vi "VP_RT_standard.vi"() -> ()   [LabVIEW 2015]
uses:
  State Enum.ctl
  Command Enum.ctl
  <vilib>/Platform/TimedLoop/XDataNode/timing_clust.ctl
  <vilib>/Platform/TimedLoop/XDataNode/nitl_modes.ctl
  <vilib>/Platform/TimedLoop/XDataNode/wakeup.ctl
  Data Write Control.ctl
  <vilib>/FPGAPlugInAG/cRIO-9039/niLvFpga_Open_cRIO-9039.vi
  <vilib>/rvi/interface/common/dynamic/niFpgaDynamicAddResources.vi
  <vilib>/Utility/error.llb/Error Cluster From Error Code.vi
  <vilib>/rvi/errors/niLvFpgaAdjustHostInterfaceError.vi
  <vilib>/rvi/interface/common/niFpgaWaitOnOcc.vi
  <vilib>/FPGAPlugInAG/Dynamic/niLvFpga_Reset_Dynamic.vi
  <vilib>/FPGAPlugInAG/Dynamic/niLvFpga_Abort_Dynamic.vi
  <vilib>/FPGAPlugInAG/Dynamic/niLvFpga_Close_Dynamic.vi
  <vilib>/Platform/TimedLoop/XDataNode/XDataNode.xnode
  <vilib>/rvi/interface/nirviOpenFPGA/nirviOpenFPGA.xnode
  FPGA Bitfiles/VP_NP_FPGA_Full.lvbitx
  <vilib>/rvi/interface/nirviReadWriteControl/nirviReadWriteControl.xnode
  <vilib>/rvi/interface/nirviMethod/nirviMethod.xnode
  <vilib>/rvi/interface/nirviCloseFPGA/nirviCloseFPGA.xnode
  <vilib>/Platform/TimedLoop/XDataNode/XDNodeRunTimeDep.lvlib
  <vilib>/rvi/errors/niLvFpgaMergeErrorWithErrorCode.vi
  NiFpgaLv.dll
  <vilib>/rvi/interface/Simulation/niFpgaSimulationCallBeginRW.vi
  <vilib>/rvi/Analysis/host/Public/NI_FpgaMspHost.lvlib
  <vilib>/FPGAPlugInAG/Dynamic/niLvFpga_StopFifo_Dynamic.vi
  <vilib>/FPGAPlugInAG/Dynamic/niLvFpga_ReadFifo_Dynamic.vi
  <vilib>/NI_Real-Time Target Support.lvlib
  <vilib>/FPGAPlugInAG/Dynamic/niLvFpga_ConfigureFifo_Dynamic.vi
panel:
  out "Z-Stage Input In Range?":bool=TRUE
  out "Y-Stage Input In Range?":bool=TRUE
  out "X-Stage Input In Range?":bool=TRUE
  in  "Tab Control":T1(tab)
  out "Fly Scan Complete":bool
  out "XY actual":cluster{"Array":dbl[], "Array":dbl[]}(graph)
  out "XY Ref":cluster{"Array":dbl[], "Array":dbl[]}(graph)
  out "Elements Available in FIFO":u32(graph)
  out "Elements Remaining in FIFO":u32(graph)
  out "Reference and Actual positions":cluster{"t0":dbl, dbl, dbl[][]}(graph)
  in  "Timeout FPGA FIFO1":i32=40000000
  out "FIFO Timed Out":bool
  out "stop case":bool
  in  "Datalog Cases":T2(ring)=enum."Data Log 16"
  out "FIFO Timed Out?":bool
  in  "FIFO Time Period":dbl=0.01 format="%#_13g"
  out "Number of Elements":u32=1250
  out "Datalog Rate (Hz)":dbl=25000.000000000004
  out "Elements Remaining":u32
  in  "Timeout (ms)":i32=10000
  out "Actual Depth":u32=131068416
  in  "Requested Depth":u32=131068000
  out "2iddVELO:VP:X_End_nm":dbl=2000.0
  out "2iddVELO:VP:X_Start_nm":dbl=-2000.0
  out "2iddVELO:VP:Start_Scan":bool
  out "2iddVELO:VP:Y_Start_nm":dbl=2000.0
  out "2iddVELO:VP:Y_End_nm":dbl=-2000.0
  out "2iddVELO:VP:Y_Step_Size_nm":dbl=50.0
  out "2iddVELO:VP:X_Step_Size_nm":dbl=50.0
  out "2iddVELO:VP:Trigger_Freq_Hz":dbl=1000.0
  out "2iddVELO:VP:Trig_DutyCycle_Per":dbl=99.0
  out "Iteration Duration RT Timed-Loop":i64=128
  in  "X Ramp Start (nm)":fxp<+/-,16,16>=-500.0
  in  "X Ramp End (nm)":fxp<+/-,16,16>=500.0
  in  "X Start Marker (nm)":fxp<+/-,58,25>
  in  "Y Ramp Start (nm)":fxp<+/-,16,16>=500.0
  in  "Y Ramp End (nm)":fxp<+/-,16,16>=-500.0
  in  "Y Step Size (nm)":fxp<+/-,16,16>=50.0
  in  "Y Start Marker (nm)":fxp<+/-,58,25>
  out "Fly Scan Running":bool
  out "Continue Run":bool
  out "X Ramp Period (usec)":fxp<+,24,24>=60000.0
  out "Y Ramp Period (usec)":fxp<+,24,24>=60000.0
  out "# of Hor Lines":fxp<+/-,34,18>=181.0 format="%.22g"
  in  "X Step Size (nm)":fxp<+/-,16,16>=50.0
  out "# of Points per Line":fxp<+/-,33,17>=180.0
  out "# Total Trigger Points":fxp<+/-,64,34>=32580.0
  out "sec per line":dbl=0.06
  out "line per sec (Hz)":dbl=16.666666666666668
  out "X Ramp Period DBL (usec)":dbl=60000.0 format="%#_6f"
  out "Total Scan Time (sec)":dbl=10.86
  in  "Controller Time Period (uSec)":u32=40
  in  "Controller Output Time Period (uSec)":u32=40
  in  "X Reference Time Period (uSec)":u32=40
  in  "Plant Output Time Period (uSec)":u32=40
  in  "Stop System (Careful!!)":bool
  in  "Datalog Time Period (uSec)":u32=40
  in  "Analog Input Time Period (uSec)":u32=40
  in  "Detector Trigger Time Period (uSec)":u32=40
  in  "Trigger Generation Time Period (uSec)":u32=40
  in  "Y Reference Time Period (uSec)":u32=40
  in  "Z Reference Time Period (uSec)":u32=40
  in  "Data Trigger Time Period (uSec)":u32=40
  in  "Reset All":bool
  in  "System Loop Type":enum16{"Open Loop", "Closed Loop"}(ring)
  in  "Base name":string="base_name"
  out "Trigger for Data":fxp<+/-,58,25>=1.0
  out "Data":fxp<+/-,58,25>[](array[numeric])
  out "Number of Data Strings":i32=5
  out "Mod6/DIO3":bool
  out "Mod5/DIO3":bool
  out "Mod4/DIO3":bool
  in  "Sample Z Stage Resolution (nm)":fxp<+,33,3>=0.5
  in  "Sample Y Stage Resolution (nm)":fxp<+,33,3>=0.5
  in  "Sample X Stage Resolution (nm)":fxp<+,33,3>=0.5
  in  "Optics Z Stage Resolution (nm)":fxp<+,33,3>=0.5
  in  "Optics Y Stage Resolution (nm)":fxp<+,33,3>=0.5
  in  "Optics X Stage Resolution (nm)":fxp<+,33,3>=0.5
  in  "Sample Z Reset":bool
  in  "Sample Y Reset":bool
  in  "Sample X Reset":bool
  out "Mod6/DIO2":bool
  out "Mod6/DIO1":bool
  out "Mod6/DIO0":bool=TRUE
  out "Mod5/DIO2":bool
  out "Mod5/DIO1":bool=TRUE
  out "Mod5/DIO0":bool
  out "Mod4/DIO2":bool=TRUE
  out "Mod4/DIO1":bool
  out "Mod4/DIO0":bool=TRUE
  in  "Optics Z Reset":bool
  in  "Optics Y Reset":bool
  in  "Optics X Reset":bool
  in  "Detector Trigger Lower Limit (V)":fxp<+/-,20,5>
  in  "Detector Trigger Upper Limit (V)":fxp<+/-,20,5>=5.0
  out "Detector Trigger (V)":fxp<+/-,20,5>
  out "Detector Trigger In Range?":bool=TRUE
  in  "Trigger High Period (usec)":fxp<+/-,64,45>=1250.0
  in  "Trigger Low Period (usec)":fxp<+/-,64,45>=1250.0
  in  "Trigger High Level (V)":fxp<+/-,20,5>=5.0
  in  "Trigger Low Level (V)":fxp<+/-,20,5>
  in  "Trigger Wave Generator":T3(ring)=enum."Square Wave 1"
  in  "DT Reference Amplitude (V)":fxp<+/-,40,17>=5.0
  in  "DT Reference DC Offset (V)":fxp<+/-,16,16>
  out "DT Frequency (periods/tick)":fxp<+,32,0>=7.500010542571545e-05
  out "DT Phase Offset (periods)":fxp<+,32,0>
  in  "DT Reset":bool
  out "DT Duty Cycle (periods)":fxp<+,32,0>=0.8799999998882413
  in  "DT phase offset (deg)":dbl format="%#.6g"
  in  "DT Frequency (Hz)":dbl=200.0 format="%#_6p"
  in  "DT duty cycle (%)":dbl=88.0 min=0.0 max=100.0 step=1.0
  in  "Z White Noise Seed":u32=4
  in  "Z White Noise Amplitude":u16=32767
  in  "Y White Noise Seed":u32=4
  in  "Y White Noise Amplitude":u16=32767
  in  "Z Reference Reset":bool
  in  "Y Reference Reset":bool
  in  "X Reference Reset":bool
  in  "Z Reference Wave Selection":T4(ring)=enum."Sine Wave"
  in  "X Reference Wave Selection":T5(ring)=enum."Custom Up Down Ramp"
  in  "Y Reference Wave Selection":T6(ring)=enum."Custom Ramp Wave"
  out "Z phase offset (periods)":fxp<+,32,0>
  out "Z frequency (periods/tick)":fxp<+,32,0>=1.25030055642128e-07 format="%.32g"
  in  "Z phase offset (deg)":dbl format="%#.6g"
  in  "Z frequency (Hz)":dbl=5.0 format="%#_6p"
  out "Y phase offset (periods)":fxp<+,32,0>
  out "Y frequency (periods/tick)":fxp<+,32,0>=5.005858838558197e-08 format="%.32g"
  in  "Y phase offset (deg)":dbl format="%#.6g"
  in  "Y frequency (Hz)":dbl=2.0 format="%#_6p"
  out "Z Stage Reference (nm)":fxp<+/-,58,25>
  out "Y Stage Reference (nm)":fxp<+/-,58,25>
  out "X Stage Reference (nm)":fxp<+/-,58,25>
  in  "X White Noise Seed":u32=4
  in  "X White Noise Amplitude":u16=32767
  in  "Z Reference DC Offset (nm)":fxp<+/-,15,15>
  in  "Y Reference DC Offset (nm)":fxp<+/-,16,16>
  in  "X Reference DC Offset (nm)":fxp<+/-,16,16>
  in  "Z Reference Amplitude (nm)":fxp<+/-,40,17>
  in  "Y Reference Amplitude (nm)":fxp<+/-,40,17>=100.0
  in  "X Reference Amplitude (nm)":fxp<+/-,40,17>=100.0
  out "X phase offset (periods)":fxp<+,32,0>
  out "X frequency (periods/tick)":fxp<+,32,0>=1.25030055642128e-07 format="%.32g"
  in  "X phase offset (deg)":dbl format="%#.6g"
  in  "X frequency (Hz)":dbl=5.0 format="%#_6p"
  in  "Scaling mV to V":fxp<+,33,10>=0.001000046730041504
  out "Heartbeat":bool=TRUE
  in  "System command":T7
  in  "Execute":bool
  out "Last Command Executed":T7
  in  "Optics and or Sample Stage":T8(ring)
  out "2iddVELO:VP:Fly_Scan":bool
  out "Remote Mode":bool
  in  "Fly Scan":bool
  in  "Local_Lock":bool
  out "Snake Scan Reference FPGA or EPICS":enum16{"FPGA Snake Scan", "EPICS Snake Scan"}(ring)
  out "Output filename":string
  out "Output path":path
  out "FPGA state":T9(ring)
  in  "cRIO data dir":string="/home/lvuser/natinst/data"
  out "RT Main Loop State":T10
  out "cRIO path":path
  out "Trigger Frequency (Hz)":dbl
  out "Trigger Duty Cycle (%)":dbl
  in  "Z-Stage Scaling Direction":fxp<+/-,3,3>=-1.0
  in  "Y-Stage Scaling Direction":fxp<+/-,3,3>=-1.0
  in  "Mod 3 AI2 V to nm Scaling":fxp<+,47,18>=1000.0
  in  "Mod 3 AI1 V to nm Scaling":fxp<+,47,18>=1000.0
  in  "Mod 3 AI0 V to nm Scaling":fxp<+,47,18>=1000.0
  out "PI Z-Stage Input (V)":fxp<+/-,20,5>=-0.000732421875
  out "PI Y-Stage Input (V)":fxp<+/-,20,5>=0.005584716796875
  out "PI X-Stage Input (V)":fxp<+/-,20,5>=-0.00311279296875
  in  "Z-Stage nm to V Scaling":fxp<+/-,32,12>=0.0005397796630859375
  in  "Y-Stage nm to V Scaling":fxp<+/-,32,12>=0.0014200210571289062
  in  "X-Stage Scaling Direction":fxp<+/-,3,3>=-1.0
  in  "X-Stage nm to V Scaling":fxp<+/-,32,12>=0.0005359649658203125
  in  "Controller Output Lower Limit":fxp<+/-,20,5>=-5.0
  in  "Controller Output Upper Limit":fxp<+/-,20,5>=5.0
  in  "FPGA Wait Timer (ms)":u16=50
  in  "Pre-Scan pause (ms)":u32=250
  in  "Readback Loop time between iterations (ms)":u32=10
  out "Measured Datalog Time Period (Ticks)":u32=1600
  out "Measured Datalog Loop Rate (secs)":dbl=3.9999999999999996e-05
  out "Measured Datalog Loop Rate (kHz)":dbl=25.000000000000004
  out "Measured Counter Loop Rate (secs)":dbl
  out "Measured Counter Loop Rate (MHz)":dbl=inf
  out "Measured X Reference Loop Rate (secs)":dbl=3.9999999999999996e-05
  out "Measured X Reference Loop Rate (kHz)":dbl=25.000000000000004
  out "Measured X Reference Time Period (Ticks)":u32=1600
  out "Measured Controller Loop Rate (kHz)":dbl=25.000000000000004
  out "Measured Controller Output Loop Rate (secs)":dbl=3.9999999999999996e-05
  out "Measured Controller Output Loop Rate (kHz)":dbl=25.000000000000004
  out "Measured Plant Output Loop Rate (secs)":dbl=3.9999999999999996e-05
  out "Measured Plant Output Loop Rate (kHz)":dbl=25.000000000000004
  out "Measured Controller Loop Rate (secs)":dbl=3.9999999999999996e-05
  out "Measured Controller Time Period (Ticks)":u32=1600
  out "Datalog Time Period (sec)":dbl=3.9999999999999996e-05
  out "Measured Controller Output Time Period (Ticks)":u32=1600
  out "Measured Plant Output Time Period (Ticks)":u32=1600
  out "Measured Counter Time Period (Ticks)":u32
  out "32 bit Count Optics X":i32
  out "32 bit Count Optics  Y":i32
  out "32 bit Count Optics  Z":i32
  out "32 bit Count Sample X":i32
  out "32 bit Count Sample  Y":i32=2
  out "32 bit Count Sample  Z":i32=-4
  out "Optics X Stage Displacement (nm)":fxp<+/-,58,25>=-1.0
  out "Optics Y Stage Displacement (nm)":fxp<+/-,58,25>
  out "Optics Z Stage Displacement (nm)":fxp<+/-,58,25>
  out "Sample X Stage Displacement (nm)":fxp<+/-,58,25>=-0.5
  out "Sample Y Stage Displacement (nm)":fxp<+/-,58,25>=1.5
  out "Sample Z Stage Displacement (nm)":fxp<+/-,58,25>=-1.0
  out "Measured Analog Input Time Period (Ticks)":u32=1600
  out "Measured Analog Input Loop Rate (secs)":dbl=3.9999999999999996e-05
  out "Measured Analog Input Loop Rate (kHz)":dbl=25.000000000000004
  out "Measured Detector Trigger Time Period (Ticks)":u32=1600
  out "Measured Trigger Gen Time Period (Ticks)":u32=1600
  out "Measured Y Reference Time Period (Ticks)":u32=1600
  out "Measured Z Reference Time Period (Ticks)":u32=1600
  out "Measured Y Reference Loop Rate (secs)":dbl=3.9999999999999996e-05
  out "Measured Y Reference Loop Rate (kHz)":dbl=25.000000000000004
  out "Measured Z Reference Loop Rate (secs)":dbl=3.9999999999999996e-05
  out "Measured Z Reference Loop Rate (kHz)":dbl=25.000000000000004
  out "Measured Data Trigger Time Period (Ticks)":u32=1600
  in  "file path soscoeff_xx1":path=path "C:/ni-rt/startup/2 ID D/Kxx/Kxx_1_Gxx_md_40us/Kxx_1_Gxx_matched_dow_16ord_mVpnm_cd8a3_AvTio9_X5nm_500pm_all_40us_soscof_xx1.mat"
  in  "file path sos gain SF Controller_xx1":path=path "C:/ni-rt/startup/2 ID D/Kxx/Kxx_1_Gxx_md_40us/Kxx_1_Gxx_matched_dow_16ord_mVpnm_cd8a3_AvTio9_X5nm_500pm_all_40us_soscof_xx2.mat"
  in  "file path soscoeff_yy1":path=path "C:/ni-rt/startup/2 ID D/Kyy/Kyy_trial_1_Gyy_md_40us/Kyy_trial_1_Gyy_matched_dow_8ord_mVpnm_cd8a3_AvTio9_Y5nm_500pm_all_40us_soscof_yy1.mat"
  in  "file path sos gain SF Controller_yy1":path=path "C:/ni-rt/startup/2 ID D/Kyy/Kyy_trial_1_Gyy_md_40us/Kyy_trial_1_Gyy_matched_dow_8ord_mVpnm_cd8a3_AvTio9_Y5nm_500pm_all_40us_soscof_yy2.mat"
  in  "file path soscoeff_zz1":path=path "C:/ni-rt/startup/2 ID D/Kzz/Kzz_1_Gzz_md_40us/Kzz_1_Gzz_matched_dow_29ord_mVpnm_cd8a3_AvTio9_Z5nm_500pm_all_40us_soscof_zz1.mat"
  in  "file path sos gain SF Controller_zz1":path=path "C:/ni-rt/startup/2 ID D/Kzz/Kzz_1_Gzz_md_40us/Kzz_1_Gzz_matched_dow_29ord_mVpnm_cd8a3_AvTio9_Z5nm_500pm_all_40us_soscof_zz2.mat"
  in  "file path soscoeff_yx1":path=path "C:/ni-rt/startup/2 ID D/Kxx/Kxx_1_Gxx_md_40us/allzero_mVpnm_XX_XY_XZ_YX_YY_YZ_ZX_ZY_ZZ_woffst_soscoeff1.mat"
  in  "file path sos gain SF Controller_yx1":path=path "C:/ni-rt/startup/2 ID D/Kxx/Kxx_1_Gxx_md_40us/allzero_mVpnm_XX_XY_XZ_YX_YY_YZ_ZX_ZY_ZZ_woffst_soscoeff2.mat"
  in  "file path soscoeff_zx1":path=path "C:/ni-rt/startup/2 ID D/Kxx/Kxx_1_Gxx_md_40us/allzero_mVpnm_XX_XY_XZ_YX_YY_YZ_ZX_ZY_ZZ_woffst_soscoeff1.mat"
  in  "file path sos gain SF Controller_zx1":path=path "C:/ni-rt/startup/2 ID D/Kxx/Kxx_1_Gxx_md_40us/allzero_mVpnm_XX_XY_XZ_YX_YY_YZ_ZX_ZY_ZZ_woffst_soscoeff2.mat"
  in  "file path soscoeff_xy1":path=path "C:/ni-rt/startup/2 ID D/Kxx/Kxx_1_Gxx_md_40us/allzero_mVpnm_XX_XY_XZ_YX_YY_YZ_ZX_ZY_ZZ_woffst_soscoeff1.mat"
  in  "file path sos gain SF Controller_xy1":path=path "C:/ni-rt/startup/2 ID D/Kxx/Kxx_1_Gxx_md_40us/allzero_mVpnm_XX_XY_XZ_YX_YY_YZ_ZX_ZY_ZZ_woffst_soscoeff2.mat"
  in  "file path soscoeff_zy1":path=path "C:/ni-rt/startup/2 ID D/Kxx/Kxx_1_Gxx_md_40us/allzero_mVpnm_XX_XY_XZ_YX_YY_YZ_ZX_ZY_ZZ_woffst_soscoeff1.mat"
  in  "file path sos gain SF Controller_zy1":path=path "C:/ni-rt/startup/2 ID D/Kxx/Kxx_1_Gxx_md_40us/allzero_mVpnm_XX_XY_XZ_YX_YY_YZ_ZX_ZY_ZZ_woffst_soscoeff2.mat"
  in  "file path soscoeff_xz1":path=path "C:/ni-rt/startup/2 ID D/Kxx/Kxx_1_Gxx_md_40us/allzero_mVpnm_XX_XY_XZ_YX_YY_YZ_ZX_ZY_ZZ_woffst_soscoeff1.mat"
  in  "file path sos gain SF Controller_xz1":path=path "C:/ni-rt/startup/2 ID D/Kxx/Kxx_1_Gxx_md_40us/allzero_mVpnm_XX_XY_XZ_YX_YY_YZ_ZX_ZY_ZZ_woffst_soscoeff2.mat"
  in  "file path soscoeff_yz1":path=path "C:/ni-rt/startup/2 ID D/Kxx/Kxx_1_Gxx_md_40us/allzero_mVpnm_XX_XY_XZ_YX_YY_YZ_ZX_ZY_ZZ_woffst_soscoeff1.mat"
  in  "file path sos gain SF Controller_yz1":path=path "C:/ni-rt/startup/2 ID D/Kxx/Kxx_1_Gxx_md_40us/allzero_mVpnm_XX_XY_XZ_YX_YY_YZ_ZX_ZY_ZZ_woffst_soscoeff2.mat"
  out "-a01(2) xx1c":fxp<+/-,64,9>[](array[numeric])=[0.637785025840232, 0.9924182654286198, 1.8461027816316544, 0.8635404845716299, 1.0670555456779864, 1.6350703383821101, 1.6323955588345012, 1.1102241390539636, 0.0, 0.0, 0.0, 0.0, 0.0, 0.0, 0.0, 0.0, 0.0, 0.0, 0.0, 0.0]
  out "-a02(2) xx1c":fxp<+/-,64,9>[](array[numeric])=[-0.999855815746439, -0.9676991072632725, -0.9642268720534838, -0.9446498323360957, -0.9442808087139987, -0.7547983908829242, -0.6690016013017409, -0.11027986125857198, 0.0, 0.0, 0.0, 0.0, 0.0, 0.0, 0.0, 0.0, 0.0, 0.0, 0.0, 0.0]
  out "b01(2) xx1c":fxp<+/-,64,9>[](array[numeric])=[-0.6378105164532328, -1.0062332697665268, -1.8762916543815855, -0.8616288879491845, -1.0856571140792324, -1.6862585929720944, -1.743591709663851, -0.6129835805090948, 0.0, 0.0, 0.0, 0.0, 0.0, 0.0, 0.0, 0.0, 0.0, 0.0, 0.0, 0.0]
  out "b02(2) xx1c":fxp<+/-,64,9>[](array[numeric])=[0.9999102047610771, 0.9971375605901365, 0.9926840301018772, 0.9509648854364836, 0.9563369558920378, 0.7818900462139817, 0.7642575436257291, 3.0531133177191805e-16, 0.0, 0.0, 0.0, 0.0, 0.0, 0.0, 0.0, 0.0, 0.0, 0.0, 0.0, 0.0]
  out "sos gain SF Controller xx1c":fxp<+/-,42,9>=-0.1625035791657865
  out "-a01(2) yy1c":fxp<+/-,64,9>[](array[numeric])=[1.8740229377643998, 1.3096977339382483, 1.7453886241944765, 0.2668895009727739, 0.0, 0.0, 0.0, 0.0, 0.0, 0.0, 0.0, 0.0, 0.0, 0.0, 0.0, 0.0, 0.0, 0.0, 0.0, 0.0]
  out "-a02(2) yy1c":fxp<+/-,64,9>[](array[numeric])=[-0.9732703278433918, -0.5194903821190732, -0.7453924481836136, -2.7755575615628914e-17, 0.0, 0.0, 0.0, 0.0, 0.0, 0.0, 0.0, 0.0, 0.0, 0.0, 0.0, 0.0, 0.0, 0.0, 0.0, 0.0]
  out "b01(2) yy1c":fxp<+/-,64,9>[](array[numeric])=[-1.8979173162254057, -1.8463149313261074, -1.7151162246453355, -0.006444279582847878, 0.0, 0.0, 0.0, 0.0, 0.0, 0.0, 0.0, 0.0, 0.0, 0.0, 0.0, 0.0, 0.0, 0.0, 0.0, 0.0]
  out "b02(2) yy1c":fxp<+/-,64,9>[](array[numeric])=[0.9969084979865663, 0.9421233904433339, 0.7362048104846675, 0.0, 0.0, 0.0, 0.0, 0.0, 0.0, 0.0, 0.0, 0.0, 0.0, 0.0, 0.0, 0.0, 0.0, 0.0, 0.0, 0.0]
  out "sos gain SF Controller yy1c":fxp<+/-,42,9>=-1.480983349494636
  out "-a01(2) zz1c":fxp<+/-,64,9>[](array[numeric])=[0.6242394224317618, 1.8967038692417004, 0.6659160318030806, 1.7792660019034106, 1.6870099721477447, 0.6417945190222861, 1.4838029149808185, 1.8456549628851837, 1.2189509782386598, 0.9933314517253298, 1.0158915520299678, 0.8863484387433826, 0.026837806879254994, 1.8269783715122585, 0.22448441435364225, 0.0, 0.0, 0.0, 0.0, 0.0]
  out "-a02(2) zz1c":fxp<+/-,64,9>[](array[numeric])=[-0.9983298461163967, -0.9972287452752734, -0.995744457243837, -0.9947210838396919, -0.9925914602095722, -0.9920974045271405, -0.9881915357970101, -0.9800069383591395, -0.9760641145386646, -0.9508624135515895, -0.9242774595356998, -0.655945641403593, -0.008661844724279444, -0.8269827070369743, 0.0, 0.0, 0.0, 0.0, 0.0, 0.0]
  out "b01(2) zz1c":fxp<+/-,64,9>[](array[numeric])=[-0.6245671059510156, -1.897930093390194, -0.6670970070931089, -1.7670265604573054, -1.6833314913922348, -0.6327437892303018, -1.5025901530730128, -1.8636454269915796, -1.1210694827766767, -0.9982206064398196, -1.0326369335418408, -1.1342635673267367, -1.6852506306166828, -0.9843740162364313, -1.7208456881689926e-15, 0.0, 0.0, 0.0, 0.0, 0.0]
  out "b02(2) zz1c":fxp<+/-,64,9>[](array[numeric])=[0.9973135069419645, 0.9951302056171929, 0.9993435624612031, 0.9919371251860779, 0.994931751453586, 0.9881092761723503, 0.9884874399279107, 0.9977145546300196, 0.9725302934743221, 0.9855561672767964, 0.9893454712398023, 0.846212786518208, 0.7855598927779743, 0.0978075435519738, 0.0, 0.0, 0.0, 0.0, 0.0, 0.0]
  out "sos gain SF Controller zz1c":fxp<+/-,42,9>=-0.1988595259608701
  out "-a01(2) yx1c":fxp<+/-,64,9>[](array[numeric])
  out "-a02(2) yx1c":fxp<+/-,64,9>[](array[numeric])
  out "b01(2) yx1c":fxp<+/-,64,9>[](array[numeric])
  out "b02(2) yx1c":fxp<+/-,64,9>[](array[numeric])
  out "sos gain SF Controller yx1c":fxp<+/-,42,9>
  out "-a01(2) zx1c":fxp<+/-,64,9>[](array[numeric])
  out "-a02(2) zx1c":fxp<+/-,64,9>[](array[numeric])
  out "b01(2) zx1c":fxp<+/-,64,9>[](array[numeric])
  out "b02(2) zx1c":fxp<+/-,64,9>[](array[numeric])
  out "sos gain SF Controller zx1c":fxp<+/-,42,9>
  out "-a01(2) xy1c":fxp<+/-,64,9>[](array[numeric])
  out "-a02(2) xy1c":fxp<+/-,64,9>[](array[numeric])
  out "b01(2) xy1c":fxp<+/-,64,9>[](array[numeric])
  out "b02(2) xy1c":fxp<+/-,64,9>[](array[numeric])
  out "sos gain SF Controller xy1c":fxp<+/-,42,9>
  out "-a01(2) zy1c":fxp<+/-,64,9>[](array[numeric])
  out "-a02(2) zy1c":fxp<+/-,64,9>[](array[numeric])
  out "b01(2) zy1c":fxp<+/-,64,9>[](array[numeric])
  out "b02(2) zy1c":fxp<+/-,64,9>[](array[numeric])
  out "sos gain SF Controller zy1c":fxp<+/-,42,9>
  out "-a01(2) xz1c":fxp<+/-,64,9>[](array[numeric])
  out "-a02(2) xz1c":fxp<+/-,64,9>[](array[numeric])
  out "b01(2) xz1c":fxp<+/-,64,9>[](array[numeric])
  out "b02(2) xz1c":fxp<+/-,64,9>[](array[numeric])
  out "sos gain SF Controller xz1c":fxp<+/-,42,9>
  out "-a01(2) yz1c":fxp<+/-,64,9>[](array[numeric])
  out "-a02(2) yz1c":fxp<+/-,64,9>[](array[numeric])
  out "b01(2) yz1c":fxp<+/-,64,9>[](array[numeric])
  out "b02(2) yz1c":fxp<+/-,64,9>[](array[numeric])
  out "sos gain SF Controller yz1c":fxp<+/-,42,9>
  out "error out (Sig Gen)":errorcluster
  out "FPGA error monitor":errorcluster
  out "FPGA end run error":errorcluster
  out "Timed Loop (end error)":errorcluster
  out "error out (Sig Gen) 2":errorcluster
  out "error out (Sig Gen) 3":errorcluster
  out "error out (Sig Gen) 4":errorcluster
  out "Main Loop error":errorcluster
  out "Main Loop Iterations":i32
  out "RT error":errorcluster
  out "EPICS comms error":errorcluster
  out "Readback error":errorcluster
  out "FPGA wait error":errorcluster
  out "Coeff file import error":errorcluster
  out "Readback loop Iterations":i32
  out "Command Loop Iterations":i32
  out "Heartbeat Loop Iterations":i32
  out "Reduced Array of States":T10[](array[typedef])
  out "XY Graph 3":cluster{"Array":dbl[], "Array":dbl[]}(graph)
  out "XY Graph 4":cluster{"Array":dbl[], "Array":dbl[]}(graph)
  out "2iddVELO:VP:cRIO_Command":string
  out "2iddVELO:VP:Controller_Type":string
  out "2iddVELO:VP:Scan_Type":string
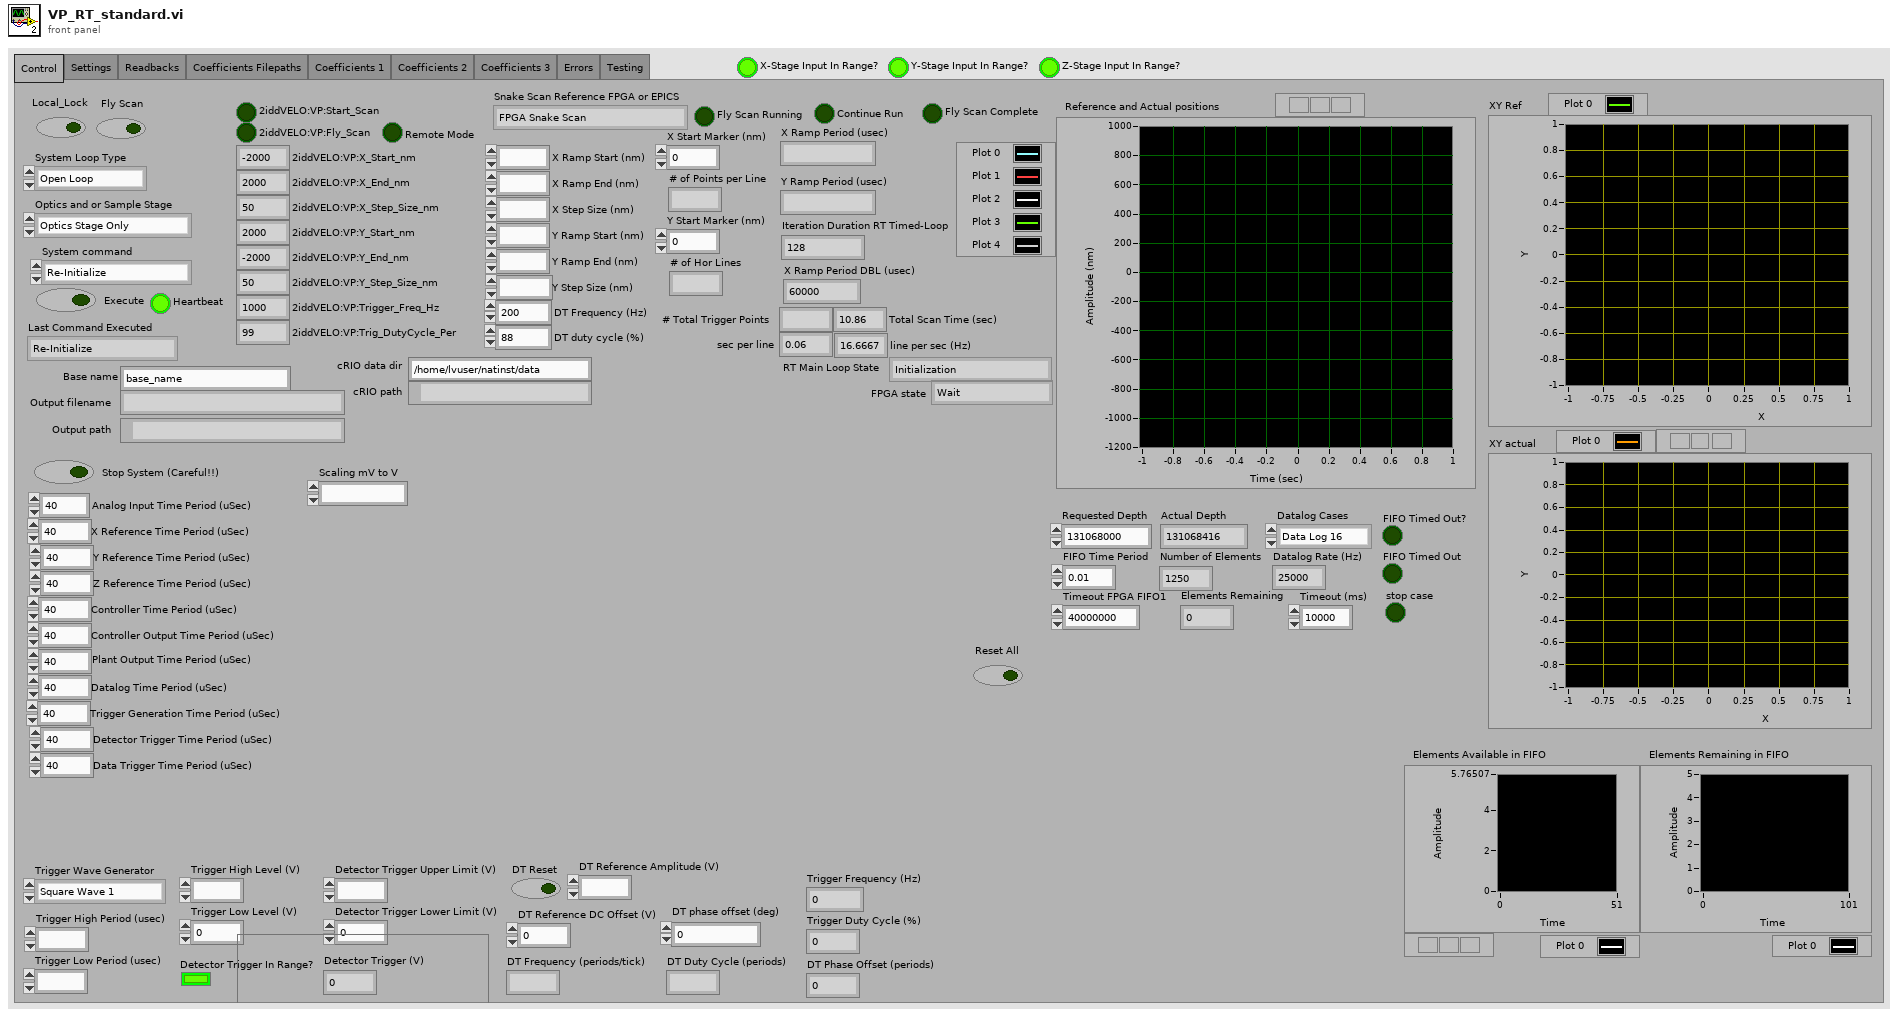
[diagram p1: front panel]
types:
  T1 = enum32{"Control", "Settings", "Readbacks", "Coefficients Filepaths", "Coefficients 1", "Coefficients 2", "Coefficients 3", "Errors", "Testing"}
  T2 = enum16{"Data Log 1", "Data Log 2", "Data Log 3", "Data Log 4", "Data Log 5", "Data Log 6", "Data Log 7", "Data Log 8", "Data Log 9", "Data Log 10", "Data Log 11", "Data Log 12", "Data Log 13", "Data Log 14", "Data Log 15", "Data Log 16"}
  T3 = enum16{"Custom Square Wave ", "Square Wave 1", "Square Wave 2"}
  T4 = enum16{"Constant", "Sine Wave", "Sawtooth Wave", "Square Wave", "Filtered White Noise"}
  T5 = enum16{"Constant", "Sine Wave", "Custom Up Down Ramp", "Filtered White Noise"}
  T6 = enum16{"Constant", "Sine Wave", "Custom Ramp Wave", "Filtered White Noise"}
  T7 = typedef "Command Enum.ctl" = enum16{"Re-Initialize ", "Update Scan Settings", "Scan", "Stop Scan", "Restart FPGA", "Stop System"}
  T8 = enum16{"Optics Stage Only", "Optics and Sample Stage"}
  T9 = enum16{"Wait", "Start Run", "Run", "End Run", "Shutdown"}
  T10 = typedef "State Enum.ctl" = enum16{"Initialization", "Import Controller coeffs", "Update Controller Info", "Wait", "Update Reference Info", "Update Detector Trigger Info", "Update Datalog Info", "Check FPGA Status", "Pre-Scan", "Start Scan", "Scanning", "End Scan", "Restart FPGA", "Stop FPGA"}
  T11 = typedef "XDNodeRunTimeDep.lvlib/timing_clust.ctl" = cluster{"Expected End [f-1]":u64, "Actual End [f-1]":u64, "Finished Late? [f-1]":bool, "Expected End [i-1]":u64, "Actual End [i-1]":u64, "Finished Late? [i-1]":bool, "Expected Start [i]":u64, "Actual Start [i]":u64, "Expected Start [f]":u64, "Actual Start [f]":u64, "Source Name":string, "Structure Name":string, "Period":i64, "Deadline":i64, "Offset":i64, "Start":i64, "Priority":i32, "Timeout":i32, "Mode":T12, "Wakeup Reason":T13, "Error":errorcluster, "Source Type":string, "Secondary Source Type":string, "Global End Time":u64, "Global Start Time":u64, "Frame Duration":u64, "Iteration Duration":u64, "Assigned CPU":i32, "I/O Scan Engine Mode":u32}
  T12 = typedef "XDNodeRunTimeDep.lvlib/nitl_modes.ctl" = enum32{"No Change", "Process missed periods, maintain original phase", "Discard missed periods, maintain original phase", "Process missed periods, ignore original phase", "Discard missed periods, ignore original phase"}
  T13 = typedef "XDNodeRunTimeDep.lvlib/wakeup.ctl" = enum32{"Normal", "Aborted", "Asynchronous wakeup", "Timing source error", "Timed loop error", "Timeout"}
  T14 = typedef "Data Write Control.ctl" = enum16{"Initialize", "Read", "Write", "Close"}
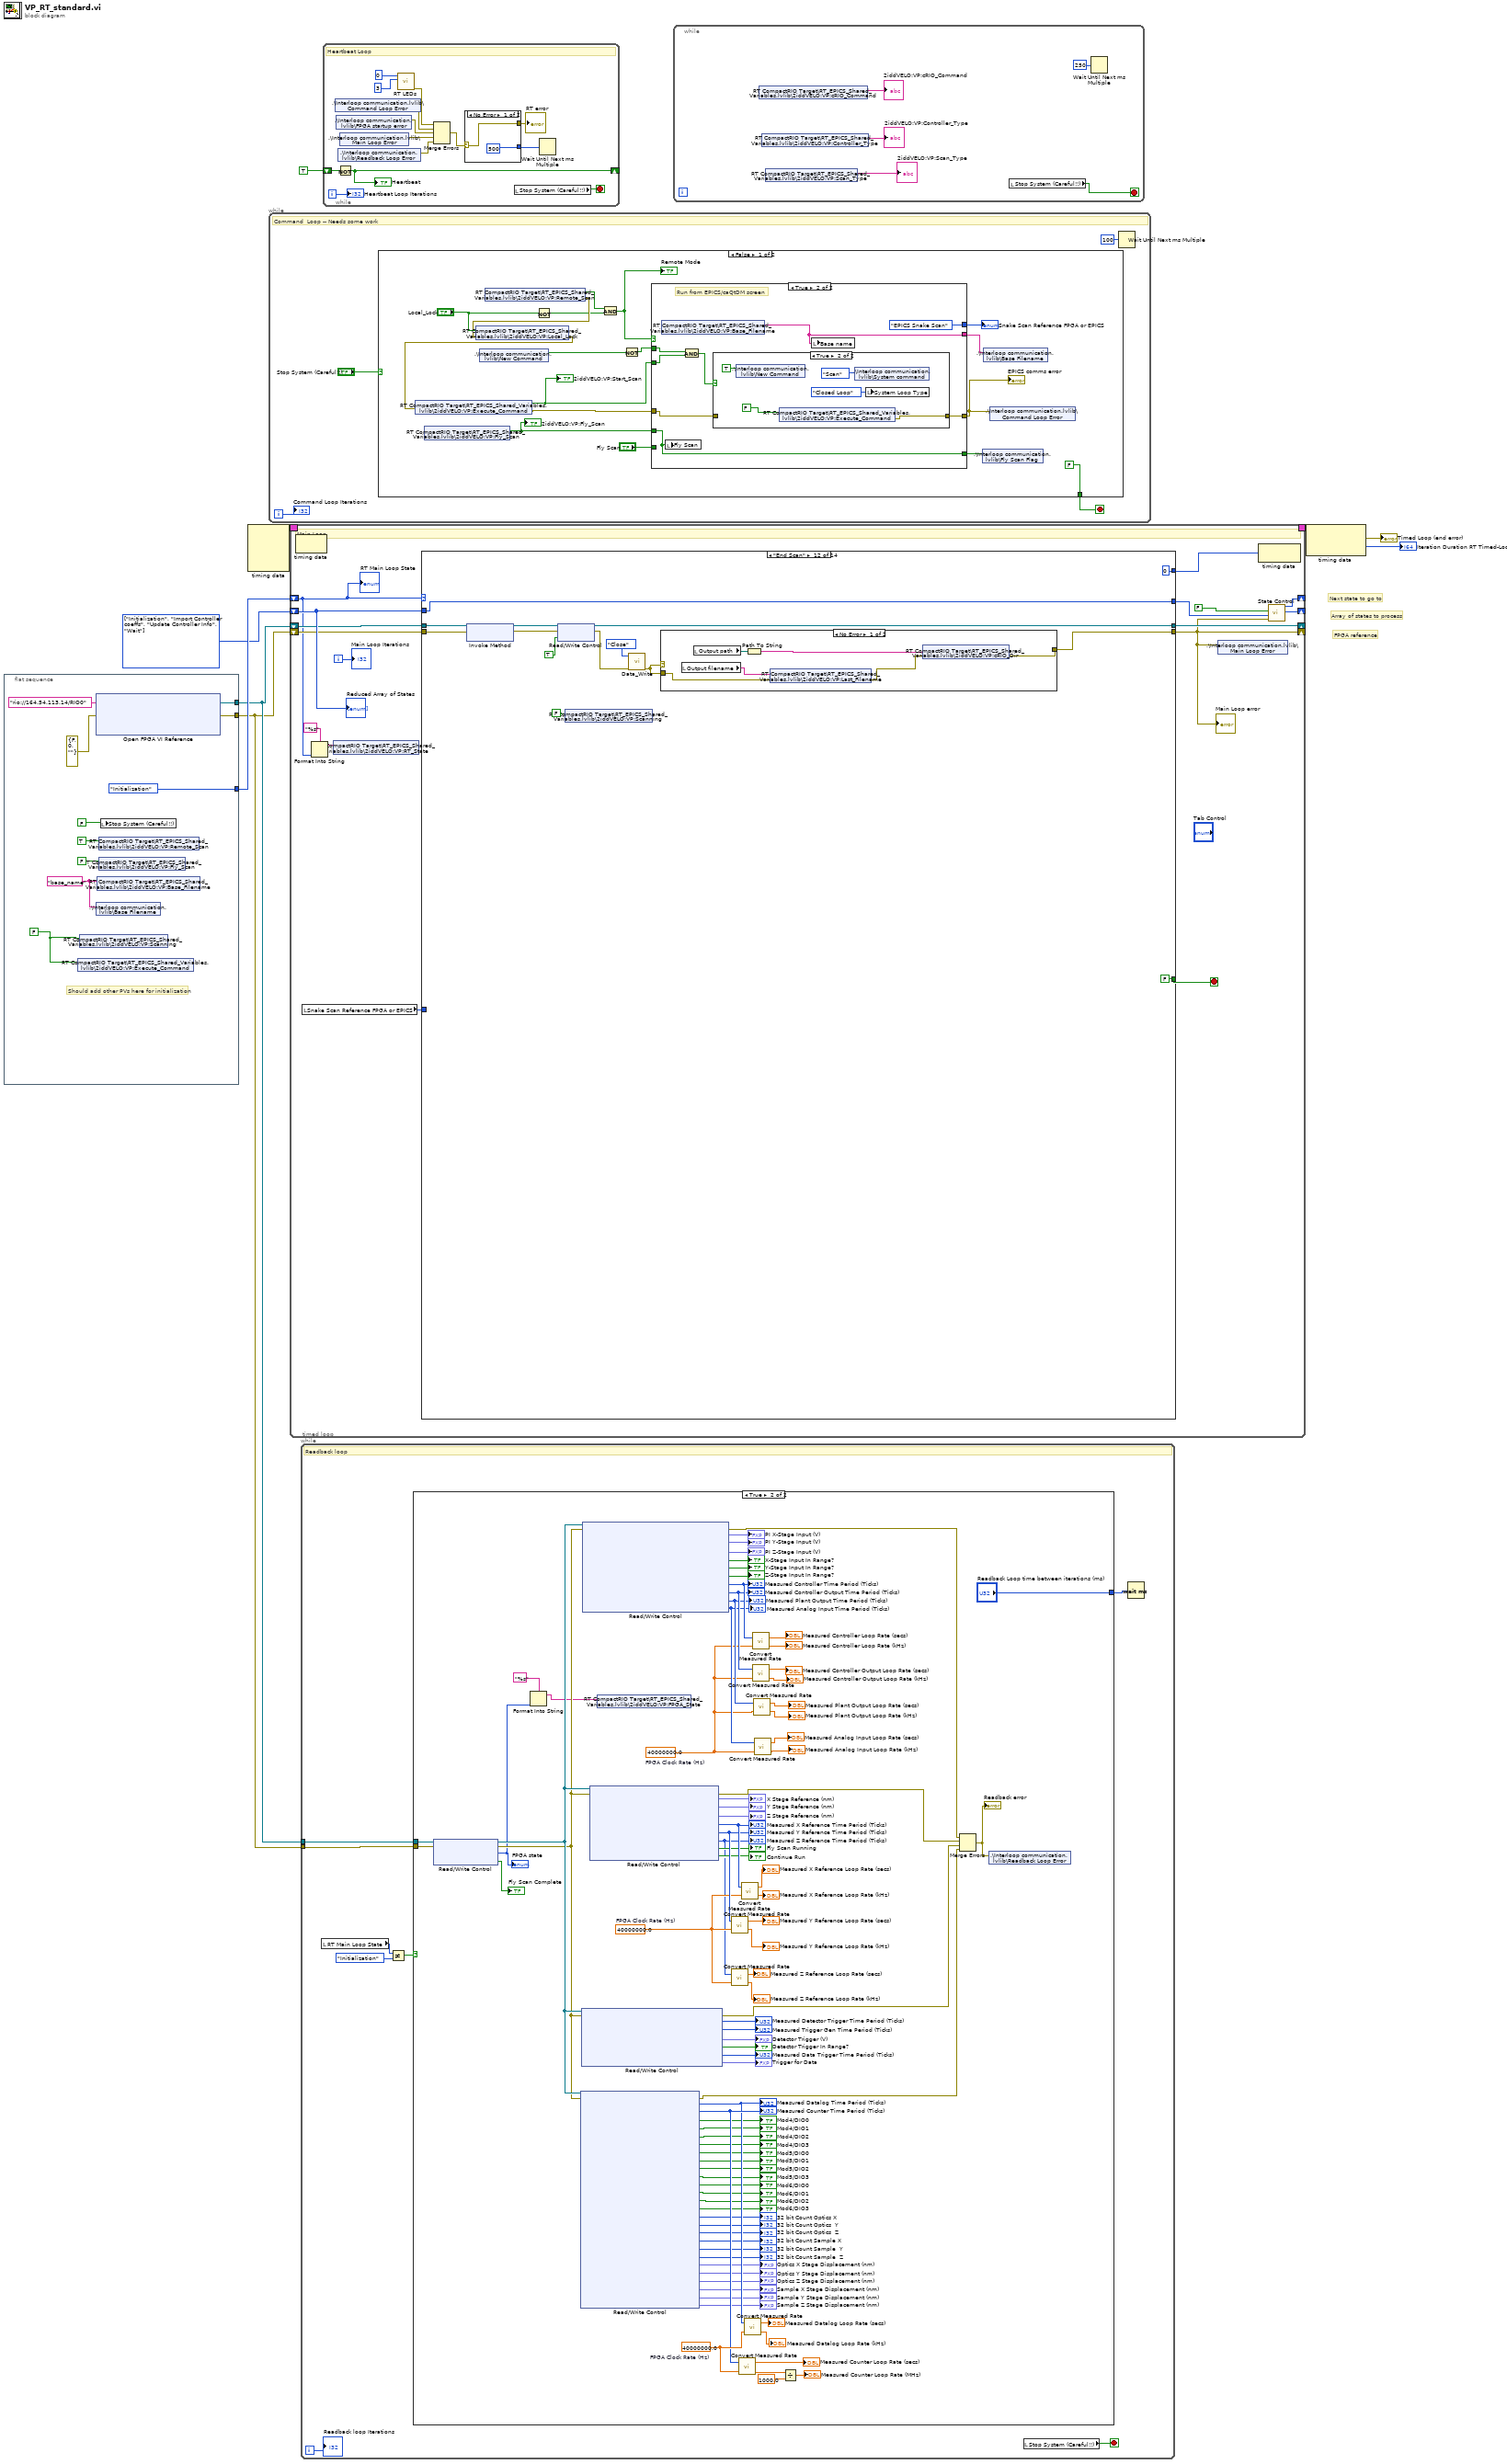
[diagram p0: block diagram]
diagram:
  w3 = T10[] [enum."Initialization", enum."Import Controller coeffs", enum."Update Controller Info", enum."Wait"] items=["Initialization", "Import Controller coeffs", "Update Controller Info", "Wait", "Update Reference Info", "Update Detector Trigger Info", "Update Datalog Info", "Check FPGA Status", "Pre-Scan", "Start Scan", "Scanning", "End Scan", "Restart FPGA", "Stop FPGA"] ("Reduced Array of States")
  # "FPGA reference"
  # "Array of states to process"
  # "Next state to go to"
  n1 = flat-sequence {
    tunnel: [State_Enum."Initialization" ("States")] -> w4
    tunnel: [w16] -> w1
    tunnel: [w15] -> w2
    frame #0 {
      w10 = FALSE ("Start_Scan")
      w13 = "base_name" ("Base_Filename")
      # "Should add other PVs here for initialization"
      n2 = shared-variable "RT CompactRIO Target\\RT_EPICS_Shared_Variables.lvlib\\2iddVELO:VP:Execute_Command"(w10) -> ()  [unwired: 1 in, 1 out]
      n3 = shared-variable "RT CompactRIO Target\\RT_EPICS_Shared_Variables.lvlib\\2iddVELO:VP:Scanning"(w10) -> ()  [unwired: 1 in, 1 out]
      n4 = xnode ("Open FPGA VI Reference")("error in"=errorcluster {"status"=FALSE, "code"=0, "source"=""} ("error constant"), "resource name"=tag "rio://164.54.113.14/RIO0") -> ("FPGA VI Reference Out"=w15:refnum<k20>, "error out"=w16:errorcluster)
      n5 = shared-variable ".\\Interloop communication.lvlib\\Base Filename"(w13) -> ()  [unwired: 1 in, 1 out]
      n6 = shared-variable "RT CompactRIO Target\\RT_EPICS_Shared_Variables.lvlib\\2iddVELO:VP:Base_Filename"(w13) -> ()  [unwired: 1 in, 1 out]
      n7 = shared-variable "RT CompactRIO Target\\RT_EPICS_Shared_Variables.lvlib\\2iddVELO:VP:Remote_Scan"(TRUE ("Remote_Scan")) -> ()  [unwired: 1 in, 1 out]
      n8 = shared-variable "RT CompactRIO Target\\RT_EPICS_Shared_Variables.lvlib\\2iddVELO:VP:Fly_Scan"(FALSE ("Fly_Scan")) -> ()  [unwired: 1 in, 1 out]
      n9 = local write "Stop System (Careful!!)"(FALSE ("Stop")) -> ()
    }
  }
  n10 = node-c288() -> (w9:T11)  [unwired: 4 in]
  n11 = while {
    i -> [w20]
    stop <- w21 stop-if-true
    # "Command  Loop -- Needs some work"
    n12 = case shown="False" "Stop System (Careful!!)" {
      tunnel: [FALSE TRUE] -> w21
      frame False {
        n13 = shared-variable "RT CompactRIO Target\\RT_EPICS_Shared_Variables.lvlib\\2iddVELO:VP:Fly_Scan"() -> (w29:bool)  [unwired: 1 in, 1 out]
        "2iddVELO:VP:Fly_Scan" <- w29
        n14 = shared-variable ".\\Interloop communication.lvlib\\New Command"() -> (w40:bool)  [unwired: 1 in, 1 out]
        n15 = shared-variable "RT CompactRIO Target\\RT_EPICS_Shared_Variables.lvlib\\2iddVELO:VP:Remote_Scan"() -> (w36:bool, error out=w34:errorcluster)  [unwired: 1 in]
        n16 = shared-variable "RT CompactRIO Target\\RT_EPICS_Shared_Variables.lvlib\\2iddVELO:VP:Local_Lock"("Local_Lock", error in=w34) -> (error out=w26:errorcluster)
        n17 = shared-variable "RT CompactRIO Target\\RT_EPICS_Shared_Variables.lvlib\\2iddVELO:VP:Execute_Command"(error in=w26) -> (w25:bool, error out=w24:errorcluster)
        "2iddVELO:VP:Start_Scan" <- w25
        n18 = Not(x="Local_Lock") -> (.not. x?=w31:bool)
        n19 = And(x=w36, y=w31) -> (x .and. y?=w37:bool)
        "Remote Mode" <- w37
        n20 = Not(x=w40) -> (.not. x?=w39:bool)
        n21 = case shown="True" w37 {
          tunnel: w25 -> [_ w57]
          tunnel: w39 -> [w48 w58]
          tunnel: [enum16{"FPGA Snake Scan", "EPICS Snake Scan"}."FPGA Snake Scan" ("Snake Scan Reference FPGA or EPICS") enum16{"FPGA Snake Scan", "EPICS Snake Scan"}."EPICS Snake Scan" ("Snake Scan Reference FPGA or EPICS")] -> w38
          tunnel: w24 -> [w42 w53]
          tunnel: [w41 w55] -> w33
          tunnel: ["Base name" w54] -> w30
          tunnel: w29 -> [_ w52]
          tunnel: [w43 w52] -> w28
          tunnel: "Fly Scan" -> [w43 _]
          frame False {
            # "Run in local mode"
            n22 = And(x="Execute", y=w48) -> (x .and. y?=w45:bool)
            n23 = shared-variable "RT CompactRIO Target\\RT_EPICS_Shared_Variables.lvlib\\2iddVELO:VP:Fly_Scan"(w43, error in=w42) -> (error out=w41:errorcluster)
            n24 = case shown="True" w45 {
              frame False {
              }
              frame True {
                n25 = shared-variable ".\\Interloop communication.lvlib\\New Command"(TRUE ("New Command")) -> ()  [unwired: 1 in, 1 out]
                n26 = shared-variable ".\\Interloop communication.lvlib\\System command"("System command") -> ()  [unwired: 1 in, 1 out]
                n27 = local write "Execute"(FALSE ("Execute")) -> ()
              }
            }
          }
          frame True {
            # "Run from EPICS/caQtDM screen"
            n28 = shared-variable "RT CompactRIO Target\\RT_EPICS_Shared_Variables.lvlib\\2iddVELO:VP:Base_Filename"() -> (w54:string)  [unwired: 1 in, 1 out]
            n29 = local write "Fly Scan"(w52) -> ()
            n30 = And(x=w58, y=w57) -> (x .and. y?=w56:bool)
            n31 = case shown="True" w56 {
              tunnel: [w60 w61] -> w55
              tunnel: w53 -> [w60 _]
              frame False {
              }
              frame True {
                n32 = shared-variable ".\\Interloop communication.lvlib\\New Command"(TRUE ("New Command")) -> ()  [unwired: 1 in, 1 out]
                n33 = shared-variable "RT CompactRIO Target\\RT_EPICS_Shared_Variables.lvlib\\2iddVELO:VP:Execute_Command"(FALSE ("2iddVELO:VP:Flyscan_Start")) -> (error out=w61:errorcluster)  [unwired: 1 in]
                n34 = shared-variable ".\\Interloop communication.lvlib\\System command"(Command_Enum."Scan" ("System command")) -> ()  [unwired: 1 in, 1 out]
                n35 = local write "System Loop Type"(enum16{"Open Loop", "Closed Loop"}."Closed Loop" ("System Loop Type")) -> ()
              }
            }
            n36 = local write "Base name"(w54) -> ()
          }
        }
        "Snake Scan Reference FPGA or EPICS" <- w38
        "EPICS comms error" <- w33
        n37 = shared-variable ".\\Interloop communication.lvlib\\Fly Scan Flag"(w28) -> ()  [unwired: 1 in, 1 out]
        n38 = shared-variable ".\\Interloop communication.lvlib\\Base Filename"(w30) -> ()  [unwired: 1 in, 1 out]
        n39 = shared-variable ".\\Interloop communication.lvlib\\Command Loop Error"(w33) -> ()  [unwired: 1 in, 1 out]